vi "UHR-Fleezers Control (host) - 10.0.vi"() -> ()   [LabVIEW 2009] (continued)
        n1548 = Multiply(x=w7137, y=w7138) -> (x*y=w7136:dbl)
        n1549 = Divide(x=w7133, y=w7139) -> (x/y=w7132:dbl)
        n1550 = Divide(x=w7136, y=w7139) -> (x/y=w7135:dbl)
        n1551 = To Word Integer(number=w7132) -> (16bit integer=w7140:i16)
        n1552 = To Word Integer(number=w7135) -> (16bit integer=w7141:i16)
        n1553 = xnode "Read/Write Control"("FPGA VI Reference In"=w7131, "error in"=w7130, "AO1"=w7140, "AO2"=w7141) -> ("error out"=w7129:errorcluster)  [unwired: 1 out]
      }
      event #40 {
        n1554 = local read "Chemyx Syringe Pump Serial Port"() -> (w7197:refnum<visa-resource-name>)
        n1555 = event-data() -> ()  [unwired: 7 out]
        n1556 = local read "Pump write delay (ms)"() -> (w7198:dbl)
        n1557 = case shown="True" "Inject Pump 1" {
          tunnel: w7198 -> [w7205 w7219]
          tunnel: w7197 -> [w7202 w7218]
          frame #0 {
            n1558 = flat-sequence {
              tunnel: w7202 -> [w7206]
              tunnel: [w7206] -> w7203
              tunnel: w7205 -> [_]
              tunnel: [w7209] -> w7204
              tunnel: w7203 -> [w7209]
              tunnel: w7204 -> [w7210]
              tunnel: [w7210] -> w7200
              tunnel: [w7212] -> w7201
              tunnel: w7200 -> [w7212]
              tunnel: w7201 -> [w7214]
              frame #0 {
                n1559 = call "Write to pump.vi"("string"="enter pump1", "VISA resource name"=w7206) -> ()  [unwired: 1 out]
              }
              frame #1 {
                n1560 = Wait (ms)(milliseconds to wait="Pump pause delay (ms)") -> ()  [unwired: 1 out]
              }
              frame #2 {
                n1561 = call "Write to pump.vi"("string"="stop", "VISA resource name"=w7210) -> ()  [unwired: 1 out]
              }
              frame #3 {
                n1562 = Wait (ms)(milliseconds to wait=u32 500) -> ()  [unwired: 1 out]
              }
              frame #4 {
                n1563 = call "Write to pump.vi"("string"="stop", "VISA resource name"=w7214) -> ()  [unwired: 1 out]
              }
            }
          }
          frame #1 {
            n1564 = flat-sequence {
              tunnel: w7218 -> [w7228]
              tunnel: w7219 -> [w7223]
              tunnel: w7219 -> [w7230]
              tunnel: w7218 -> [w7231]
              tunnel: [w7231] -> w7216
              tunnel: [w7233] -> w7217
              tunnel: w7216 -> [w7233]
              tunnel: w7217 -> [w7235]
              frame #0 {
                n1565 = local read "All Pump Parameters"() -> (w7222:T5)
                n1566 = Unbundle By Name(w7222) -> ("Pump 1"=w7229:T45)
                n1567 = call "Set pump parameters.vi"("Pump write delay (ms)"=w7223, "Volume (uL)"="Ch 2 Inject Volume (uL)", "Rate (uL/h)"="Ch 1 Inject Rate (ul/h)", "Units"=4.0, "Pump #"=1.0, "Pump Parameters In"=w7229, "VISA resource name"=w7228) -> ("Pump Parameters Out"=w7221:T45)  [unwired: 3 in]
                n1568 = Bundle By Name(cluster=w7222, "Pump 1"=w7221) -> (w7220:T5)
                n1569 = local write "All Pump Parameters"(w7220) -> ()
              }
              frame #1 {
                n1570 = Wait (ms)(milliseconds to wait=w7230) -> ()  [unwired: 1 out]
              }
              frame #2 {
                n1571 = call "Write to pump.vi"("string"="start", "VISA resource name"=w7231) -> ()  [unwired: 1 out]
              }
              frame #3 {
                n1572 = Wait (ms)(milliseconds to wait=u32 500) -> ()  [unwired: 1 out]
              }
              frame #4 {
                n1573 = call "Write to pump.vi"("string"="start", "VISA resource name"=w7235) -> ()  [unwired: 1 out]
              }
            }
          }
        }
      }
      event #41 {
        n1574 = event-data() -> ()  [unwired: 7 out]
        n1575 = local read "Pump write delay (ms)"() -> (w7238:dbl)
        n1576 = case shown="False" "Inject Pump 3" {
          tunnel: w7238 -> [w7245 w7259]
          tunnel: "Chemyx Syringe Pump Serial Port" -> [w7242 w7258]
          frame #0 {
            n1577 = flat-sequence {
              tunnel: w7242 -> [w7246]
              tunnel: [w7246] -> w7243
              tunnel: w7245 -> [_]
              tunnel: [w7249] -> w7244
              tunnel: w7243 -> [w7249]
              tunnel: w7244 -> [w7250]
              tunnel: [w7250] -> w7240
              tunnel: [w7252] -> w7241
              tunnel: w7240 -> [w7252]
              tunnel: w7241 -> [w7254]
              frame #0 {
                n1578 = call "Write to pump.vi"("string"="enter pump3", "VISA resource name"=w7246) -> ()  [unwired: 1 out]
              }
              frame #1 {
                n1579 = local read "Pump pause delay (ms)"() -> (w7248:u32)
                n1580 = Wait (ms)(milliseconds to wait=w7248) -> ()  [unwired: 1 out]
              }
              frame #2 {
                n1581 = call "Write to pump.vi"("string"="stop", "VISA resource name"=w7250) -> ()  [unwired: 1 out]
              }
              frame #3 {
                n1582 = Wait (ms)(milliseconds to wait=u32 0) -> ()  [unwired: 1 out]
              }
              frame #4 {
                n1583 = call "Write to pump.vi"("string"="stop", "VISA resource name"=w7254) -> ()  [unwired: 1 out]
              }
            }
          }
          frame #1 {
            n1584 = flat-sequence {
              tunnel: w7258 -> [w7268]
              tunnel: w7259 -> [w7263]
              tunnel: w7259 -> [w7270]
              tunnel: w7258 -> [w7271]
              tunnel: [w7271] -> w7256
              tunnel: [w7274] -> w7257
              tunnel: w7256 -> [w7274]
              tunnel: w7257 -> [w7275]
              frame #0 {
                n1585 = local read "All Pump Parameters"() -> (w7262:T5)
                n1586 = Unbundle By Name(w7262) -> ("Pump 3"=w7269:T45)
                n1587 = call "Set pump parameters.vi"("Pump write delay (ms)"=w7263, "Volume (uL)"="Ch 3 Inject Volume (uL)", "Rate (uL/h)"="Ch 3 Inject Rate (ul/h)", "Units"=4.0, "Pump #"=3.0, "Pump Parameters In"=w7269, "VISA resource name"=w7268) -> ("Pump Parameters Out"=w7261:T45)  [unwired: 3 in]
                n1588 = Bundle By Name(cluster=w7262, "Pump 3"=w7261) -> (w7260:T5)
                n1589 = local write "All Pump Parameters"(w7260) -> ()
              }
              frame #1 {
                n1590 = Wait (ms)(milliseconds to wait=w7270) -> ()  [unwired: 1 out]
              }
              frame #2 {
                n1591 = call "Write to pump.vi"("string"="start", "VISA resource name"=w7271) -> ()  [unwired: 1 out]
              }
              frame #3 {
                n1592 = Wait (ms)(milliseconds to wait=u32 500) -> ()  [unwired: 1 out]
              }
              frame #4 {
                n1593 = call "Write to pump.vi"("string"="start", "VISA resource name"=w7275) -> ()  [unwired: 1 out]
              }
            }
          }
        }
      }
      event #42 {
        n1594 = event-data() -> ()  [unwired: 7 out]
        n1595 = local read "Pump write delay (ms)"() -> (w7279:dbl)
        n1596 = flat-sequence {
          tunnel: w7277 -> [w7292]
          tunnel: w7279 -> [w7288]
          tunnel: "Inject Pump 2" -> [_]
          tunnel: w7279 -> [w7294]
          tunnel: w7277 -> [w7295]
          frame #0 {
            n1597 = local read "All Pump Parameters"() -> (w7287:T5)
            n1598 = Multiply(x=60.0, y="Flush Center Ch Rate (ul/m)") -> (x*y=w7284:dbl)
            n1599 = Unbundle By Name(w7287) -> ("Pump 2"=w7293:T45)
            n1600 = call "Set pump parameters.vi"("Pump write delay (ms)"=w7288, "Volume (uL)"="Flush Center Ch Volume (uL)", "Rate (uL/h)"=w7284, "Units"=3.0, "Pump #"=2.0, "Pump Parameters In"=w7293, "VISA resource name"=w7292) -> ("Pump Parameters Out"=w7286:T45)  [unwired: 3 in]
            n1601 = Bundle By Name(cluster=w7287, "Pump 2"=w7286) -> (w7285:T5)
            n1602 = local write "All Pump Parameters"(w7285) -> ()
            n1603 = Add(x="Flush Center Ch Volume (uL)", y="Total Volume\nFlushed (uL)") -> (x+y=w7281:dbl)
            n1604 = local write "Total Volume\nFlushed (uL)"(w7281) -> ()
          }
          frame #1 {
            n1605 = Wait (ms)(milliseconds to wait=w7294) -> ()  [unwired: 1 out]
          }
          frame #2 {
            n1606 = call "Write to pump.vi"("string"="start", "VISA resource name"=w7295) -> ()  [unwired: 1 out]
          }
        }
        n1607 = local read "Chemyx Syringe Pump Serial Port"() -> (w7277:refnum<visa-resource-name>)
      }
      event #43 {
        n1608 = event-data() -> ()  [unwired: 7 out]
        n1609 = Select(t="run" ("string"), s="Sample Channel Flow", f="stop" ("string")) -> (s? t:f=w7297:string)
        n1610 = Concatenate Strings(w7297, "\r") -> (w7301:string)
        n1611 = VISA Write(VISA resource name=w7303, write buffer=w7301) -> ()  [unwired: 1 in, 3 out]
      }
      event #44 {
        n1612 = event-data() -> ()  [unwired: 7 out]
        n1613 = Not(x="Flip Green Filter") -> (.not. x?=w7304:bool)
        n1614 = local write "Flip Green Filter"(w7304) -> ()
        n1615 = flat-sequence {
          tunnel: w7312 -> [w7317]
          tunnel: w7311 -> [w7316]
          tunnel: [w7314] -> w7309
          tunnel: [w7313] -> w7308
          tunnel: [w7356] -> w7307
          tunnel: w7309 -> [w7356]
          tunnel: [w7355] -> w7306
          tunnel: w7308 -> [w7355]
          tunnel: w7307 -> [w7360]
          tunnel: w7306 -> [w7359]
          tunnel: [w7358] -> w7310
          frame #0 {
            n1616 = xnode "Read/Write Control"("FPGA VI Reference In"=w7317, "error in"=w7316, "Green Filter Flipper"=TRUE) -> ("FPGA VI Reference Out"=w7314:T20, "error out"=w7313:errorcluster)
          }
          frame #1 {
            n1617 = Wait (ms)(milliseconds to wait=u32 100) -> ()  [unwired: 1 out]
          }
          frame #2 {
            n1618 = xnode "Read/Write Control"("FPGA VI Reference In"=w7360, "error in"=w7359, "Green Filter Flipper"=FALSE) -> ("error out"=w7358:errorcluster)  [unwired: 1 out]
          }
        }
      }
      event #45 {
        n1619 = event-data() -> ()  [unwired: 7 out]
        n1620 = local read "Pump 1 contents"() -> (→"Pump 1 cont disp":string)
        n1621 = local read "Pump 3 contents"() -> (→"Pump 3 cont disp":string)
      }
      event #46 {
        n1622 = event-data() -> ()  [unwired: 7 out]
        n1623 = xnode "Read/Write Control"("FPGA VI Reference In"=w7403, "error in"=w7402, "Trap Pos. FB Reset"="Reset Trap Pos. FB") -> ()  [unwired: 2 out]
      }
      event #47 {
        n1624 = event-data() -> ()  [unwired: 7 out]
        n1625 = xnode "Read/Write Control"("FPGA VI Reference In"=w7443, "error in"=w7442, "Force feedback"="Trap Pos. FB ON") -> ()  [unwired: 2 out]
      }
      event #48 {
        n1626 = event-data() -> ()  [unwired: 7 out]
        n1627 = xnode "Read/Write Control"("FPGA VI Reference In"=w7489, "error in"=w7488, "Trap Pos. FB Range"="Trap Pos. FB Range", "Trap Pos. FB Gains"="Trap Pos. FB Gains", "Trap Pos. FB Mult Factor"="Trap Pos. FB Mult Factor", "Trap Pos. FB Offset Factor"="Trap Pos. FB Offset Factor", "Trap Pos FB Negate Action"="Trap Pos FB Negate Action", "Trap Pos FB Monitor T1 or T2"="Trap Pos FB Monitor\nT1 or T2", "AI1 X Scale"="Trap Pos. AI1 X Pre-scale") -> ()  [unwired: 2 out]
      }
      event #49 {
        n1628 = event-data() -> ()  [unwired: 7 out]
        n1629 = xnode "Read/Write Control"("FPGA VI Reference In"=w7625, "error in"=w7624, "Trap Pos. FB SP"="Trap Pos FB SP") -> ()  [unwired: 2 out]
      }
      event #50 {
        n1630 = event-data() -> ()  [unwired: 7 out]
        n1631 = local read "Trap Pos FB Monitor\nT1 or T2"() -> (w7677:bool)
        n1632 = local read "Trap X AI1 (DMA)"() -> (w7680:T10)
        n1633 = local read "Trap X AI1"() -> (w7683:T10)
        n1634 = Unbundle By Name(w7683) -> ("Set 1"=w7682:fxp<+/-,16,1>, "Set 2"=w7681:fxp<+/-,16,1>)
        n1635 = Unbundle By Name(w7680) -> ("Set 1"=w7679:fxp<+/-,16,1>, "Set 2"=w7678:fxp<+/-,16,1>)
        n1636 = Select(t=w7682, s=w7677, f=w7681) -> (s? t:f=w7676:fxp<+/-,16,1>)
        n1637 = Select(t=w7679, s=w7677, f=w7678) -> (s? t:f=w7675:fxp<+/-,16,1>)
        n1638 = Not(x="Set SP Using...") -> (.not. x?=w7670:bool)
        n1639 = Select(t=w7676, s=w7670, f=w7675) -> (s? t:f=w7671:fxp<+/-,16,1>)
        n1640 = xnode "Read/Write Control"("FPGA VI Reference In"=w7673, "error in"=w7672, "Trap Pos. FB SP"=w7671) -> ()  [unwired: 2 out]
        n1641 = local write "Trap Pos FB SP"(w7671) -> ()
      }
      event #51 {
        n1642 = event-data() -> ()  [unwired: 7 out]
        n1643 = Scale By Power Of 2(n="Trap Pos. FB Out Scale 2^n", x=ext 1.0) -> (x*2^n=w7729:ext)
        n1644 = property on="Trap Pos. FB Mult Factor" class="DigNum (strict)"("Val(Sgnl)"=w7729) -> ()  [unwired: 2 in, 2 out]
      }
    }
    "error out 2" <- w4459
    n1645 = node-c288() -> ()  [unwired: 2 out]
  }
  n1646 = timed-loop "Oscillate AOD (debugging)" {
    tunnel: w14 -> [w7733]
    tunnel: [w7732] -> w55
    timing: w50 -> [_]
    timing-out: [_] -> w49
    stop <- w7732 stop-if-true
    n1647 = node-c288() -> ()  [unwired: 2 out]
    n1648 = event shown="[0] \"Oscillate Set 1\", \"Fish for Tether\": Value Change" {
      selector: _ -> [_ _ _]
      dyn-events: _ -> [_ _ _]
      timeout: _ -> [_ _ _]
      tunnel: w7733 -> [w7740 _ _]
      tunnel: [FALSE ("Stop All") _ w7993] -> w7732
      event #0 {
        n1649 = event-data() -> ()  [unwired: 6 out]
        n1650 = local read "Oscillate Set 1"() -> (w7739:bool)
        n1651 = Or(x=w7739, y="Fish for Tether") -> (x .or. y?=w7737:bool)
        n1652 = case shown="True" w7737 {
          tunnel: w7740 -> [_ w7742]
          tunnel: "Fish for Tether" -> [_ w7741]
          frame #0 {
          }
          frame #1 {
            n1653 = case shown="True" w7741 {
              frame #0 {
              }
              frame #1 {
                n1654 = local write "Scan axis 2"(TRUE) -> ()
                n1655 = local write "Tether"(FALSE ("Tether")) -> ()
              }
            }
            n1656 = node-c288() -> (w7744:T22)  [unwired: 4 out]
            n1657 = timed-loop "Oscillate AOD" {
              timing: w7744 -> [_]
              timing-out: [_] -> w7743
              tunnel: w7742 -> [w7754]
              tunnel: w7741 -> [w7753]
              i -> [w7756]
              stop <- w7752 stop-if-true
              n1658 = node-c288() -> (w7755:i64)  [unwired: 1 out]
              n1659 = flat-sequence {
                tunnel: w7756 -> [w7783]
                tunnel: w7755 -> [w7782]
                tunnel: w7754 -> [w7761]
                tunnel: w7753 -> [w7764]
                tunnel: [w7764] -> w7751
                tunnel: [w7763] -> w7750
                tunnel: [w7760] -> w7749
                tunnel: [w7757] -> w7747
                tunnel: w7751 -> [w7819]
                tunnel: w7750 -> [w7817]
                tunnel: w7749 -> [w7816]
                tunnel: [w7815] -> w7748
                tunnel: w7747 -> [w7814]
                tunnel: [w7867] -> w7752
                tunnel: w7748 -> [w7866]
                frame #0 {
                  n1660 = Divide(x=w7782, y=i64 1000) -> (x/y=w7777:dbl)
                  n1661 = Multiply(x=w7777, y=w7783) -> (x*y=w7779:dbl)
                  n1662 = local read "BD 1 Frequency 2 (MHz)"() -> (w7762:dbl)
                  n1663 = Multiply(x="Osc. freq. (Hz)", y=6.283185307179586) -> (x*y=w7780:dbl)
                  n1664 = Multiply(x=w7780, y=w7779) -> (x*y=w7759:dbl)
                  n1665 = local read "BD 1 Frequency 1 (MHz)"() -> (w7767:dbl)
                  n1666 = case shown="True" w7764 {
                    tunnel: w7759 -> [w7789 w7794]
                    tunnel: w7767 -> [_ w7805]
                    tunnel: w7762 -> [_ w7806]
                    tunnel: [w7786 w7800] -> w7765
                    tunnel: [FALSE w7797] -> w7760
                    tunnel: [0.0 w7790] -> w7757
                    frame #0 {
                      n1667 = Sine(x=w7789) -> (sin(x)=w7787:dbl)
                      n1668 = Multiply(x=w7787, y="Osc. amp. (MHz)") -> (x*y=w7786:dbl)
                    }
                    frame #1 {
                      n1669 = Cosine(x=w7794) -> (cos(x)=w7809:dbl)
                      n1670 = Subtract(x=w7806, y=w7805) -> (x-y=w7804:dbl)
                      n1671 = Decrement(x=w7809) -> (x-1=w7808:dbl)
                      n1672 = Subtract(x=w7804, y="Closest Delta (MHz)") -> (x-y=w7801:dbl)
                      n1673 = Divide(x=w7808, y=-2.0) -> (x/y=w7802:dbl)
                      n1674 = Multiply(x=w7802, y=w7801) -> (x*y=w7800:dbl)
                      n1675 = local read "Vec Mean of T1 T2"() -> (w7796:dbl[])
                      n1676 = Greater?(x=w7796, y="Stop F (pN)") -> (0:w7798:bool[])
                      n1677 = Or Array Elements(Boolean array=w7798) -> (logical OR=w7797:bool)
                      n1678 = Divide(x=w7794, y=6.283185307179586) -> (x/y=w7793:dbl)
                      n1679 = Round Toward +Infinity(x=w7793) -> (ceil(x): smallest int >= x=w7790:dbl)
                      "Attempts" <- w7790
                      n1680 = Greater?(x=w7790, y="Attempt Limit") -> (0:w7792:bool)
                      n1681 = case shown="True" w7792 {
                        frame #0 {
                        }
                        frame #1 {
                          n1682 = call <vilib>:"Beep.vi"() -> ()  [unwired: 3 in, 9 out]
                          n1683 = local write "Fish for Tether"(FALSE ("Fish for Tether")) -> ()
                          n1684 = local read "Messages"() -> (w7811:string)
                          n1685 = call "Update messages.vi"("Message to add"="Tether fishing timeout." ("Messages"), "Old message string"=w7811) -> ("New message string"=→"Messages":string)
                        }
                      }
                    }
                  }
                  n1686 = local read "BD 2 Frequency 1 (MHz)"() -> (w7766:dbl)
                  n1687 = Select(t=w7767, s="Scan axis 2", f=w7766) -> (s? t:f=w7770:dbl)
                  n1688 = Add(x=w7765, y=w7770) -> (x+y=w7763:dbl)
                  n1689 = Select(t=w7763, s="Scan axis 2", f=w7767) -> (s? t:f=w7773:dbl)
                  n1690 = Select(t=w7766, s="Scan axis 2", f=w7763) -> (s? t:f=w7772:dbl)
                  n1691 = local read "Y RF Frequency Limits (MHz)"() -> (w7768:T15)
                  n1692 = local read "X RF Frequency Limits (MHz)"() -> (w7769:T15)
                  n1693 = local read "BD 1 Frequency 3 (MHz)"() -> (w7776:dbl)
                  n1694 = local read "BD 2 Frequency 2 (MHz)"() -> (w7775:dbl)
                  n1695 = local read "BD 2 Frequency 3 (MHz)"() -> (w7774:dbl)
                  n1696 = call "set RF board frequency - interlace.vi"("Board 2 Frequency Limits"=w7768, "Board 1 Frequency Limits"=w7769, "FPGA VI Reference In"=w7761, "Board 2 Frequency 3 (MHz)"=w7774, "Board 1 Frequency 3 (MHz)"=w7776, "Board 2 Frequency 2 (MHz)"=w7775, "Board 2 Frequency 1 (MHz)"=w7772, "Board 1 Frequency 2 (MHz)"=w7762, "Board 1 Frequency 1  (MHz)"=w7773) -> ()  [unwired: 1 in, 2 out]
                }
                frame #1 {
                  n1697 = And(x=w7819, y=w7816) -> (x .and. y?=w7818:bool)
                  n1698 = case "Only if were fishing and now formed tether" shown="True" w7818 {
                    tunnel: w7817 -> [w7821 w7834]
                    tunnel: [w7820 w7833] -> w7815
                    tunnel: w7814 -> [_ w7829]
                    frame #0 {
                      n1699 = local read "Fish for Tether"() -> (w7820:bool)
                      n1700 = case shown="False" w7820 {
                        tunnel: w7821 -> [w7822 _]
                        frame #0 {
                          n1701 = property on="BD 1 Frequency 1 (MHz)" class="DigNum (strict)"("Val(Sgnl)"=w7822) -> ()  [unwired: 2 in, 2 out]
                        }
                        frame #1 {
                        }
                      }
                    }
                    frame #1 {
                      w7833 = FALSE ("Fish for Tether")
                      n1702 = call <vilib>:"Beep.vi"() -> ()  [unwired: 3 in, 9 out]
                      n1703 = Number To Decimal String(number=w7829, width (-)=i16 1) -> (decimal integer string=w7827:string)
                      n1704 = case shown="\"2\", \"3\", \"4\", \"5\", \"6\"" "Then..." {
                        selector: "Then..." -> [_ w7837]
                        tunnel: w7834 -> [w7836 _]
                        frame #0 {
                          n1705 = property on="BD 1 Frequency 1 (MHz)" class="DigNum (strict)"("Val(Sgnl)"=w7836) -> ()  [unwired: 2 in, 2 out]
                        }
                        frame #1 {
                          n1706 = flat-sequence {
                            tunnel: w7837 -> [w7839]
                            frame #0 {
                              n1707 = property on="Trap Delta (MHz)" class="DigNum (strict)"("Val(Sgnl)"="Move to Delta 1 (MHz)") -> ()  [unwired: 2 in, 2 out]
                            }
                            frame #1 {
                              n1708 = case shown="\"5\", \"6\"" w7839 {
                                selector: w7839 -> [w7842 w7852 _]
                                frame #0 {
                                n1709 = flat-sequence {
                                tunnel: w7842 -> [w7843]
                                tunnel: [w7843] -> w7840
                                tunnel: [w7845] -> w7841
                                tunnel: w7840 -> [w7845]
                                tunnel: w7841 -> [w7849]
                                frame #0 {
                                n1710 = property on="Green Laser ON/Interlacing" class="Bool (strict)"("Val(Sgnl)"=TRUE ("Value (Signaling)")) -> ()  [unwired: 2 in, 2 out]
                                }
                                frame #1 {
                                n1711 = Multiply(x="Wait Before Save (s)", y=u32 1000 ("x")) -> (x*y=w7847:u32)
                                n1712 = Wait (ms)(milliseconds to wait=w7847) -> ()  [unwired: 1 out]
                                }
                                frame #2 {
                                n1713 = property on="Start Saving" class="Bool (strict)"("Value"=TRUE ("Start Saving")) -> ()  [unwired: 2 in, 2 out]
                                n1714 = case shown="\"4\"" w7849 {
                                frame #0 {
                                }
                                frame #1 {
                                n1715 = property on="Fl. Triggered..." class="Bool (strict)"("Val(Sgnl)"=TRUE ("Value (Signaling)")) -> ()  [unwired: 2 in, 2 out]
                                }
                                }
                                }
                                }
                                }
                                frame #1 {
                                n1716 = flat-sequence {
                                tunnel: w7852 -> [w7860]
                                frame #0 {
                                n1717 = Wait (ms)(milliseconds to wait=u32 500) -> ()  [unwired: 1 out]
                                }
                                frame #1 {
                                n1718 = property on="Trap Raster Scan" class="Bool (strict)"("Val(Sgnl)"=TRUE ("Value (Signaling)")) -> ()  [unwired: 2 in, 2 out]
                                }
                                frame #2 {
                                n1719 = Wait (ms)(milliseconds to wait=u32 500) -> ()  [unwired: 1 out]
                                }
                                frame #3 {
                                n1720 = while {
                                stop <- w7856 stop-if-true
                                n1721 = local read "Saving..."() -> (w7857:bool)
                                n1722 = Wait (ms)(milliseconds to wait=u32 100) -> ()  [unwired: 1 out]
                                n1723 = Not(x=w7857) -> (.not. x?=w7856:bool)
                                }
                                }
                                frame #4 {
                                n1724 = property on="Trap Delta (MHz)" class="DigNum (strict)"("Val(Sgnl)"="Move to Delta 2 (MHz)") -> ()  [unwired: 2 in, 2 out]
                                }
                                frame #5 {
                                n1725 = case shown="\"6\"" w7860 {
                                frame #0 {
                                }
                                frame #1 {
                                n1726 = local read "Tether"() -> (w7861:bool)
                                n1727 = case shown="True" w7861 {
                                frame #0 {
                                }
                                frame #1 {
                                n1728 = flat-sequence {
                                frame #0 {
                                n1729 = Wait (ms)(milliseconds to wait=u32 500) -> ()  [unwired: 1 out]
                                }
                                frame #1 {
                                n1730 = property on="Green Laser ON/Interlacing" class="Bool (strict)"("Val(Sgnl)"=TRUE ("Green Laser ON/Interlacing")) -> ()  [unwired: 2 in, 2 out]
                                }
                                frame #2 {
                                n1731 = Wait (ms)(milliseconds to wait=u32 500) -> ()  [unwired: 1 out]
                                }
                                frame #3 {
                                n1732 = local write "Start Saving"(TRUE ("Start Saving")) -> ()
                                }
                                }
                                }
                                }
                                }
                                }
                                }
                                }
                                }
                                frame #2 {
                                }
                              }
                            }
                          }
                        }
                      }
                      n1733 = Concatenate Strings("Formed tether in ", w7827, " attempt(s)." ("string")) -> (w7824:string)
                      n1734 = local read "Messages"() -> (w7831:string)
                      n1735 = local write "Fish for Tether"(w7833) -> ()
                      n1736 = call "Update messages.vi"("Message to add"=w7824, "Old message string"=w7831) -> ("New message string"=w7830:string)
                      n1737 = local write "Messages"(w7830) -> ()
                      n1738 = Get Date/Time In Seconds() -> (seconds since 1Jan1904=→"Time tether formed":timestamp)
                      "Tether" <- "Tether Alarm?"
                    }
                  }
                }
                frame #2 {
                  n1739 = local read "Oscillate Set 1"() -> (w7871:bool)
                  n1740 = Or(x=w7871, y=w7866) -> (x .or. y?=w7868:bool)
                  n1741 = local read "Stop All"() -> (w7869:bool)
                  n1742 = Not(x=w7868) -> (.not. x?=w7870:bool)
                  n1743 = Compound Arithmetic op=OR(w7869, w7870) -> (w7867:bool)
                }
              }
              n1744 = node-c288() -> ()  [unwired: 2 out]
            }
            n1745 = node-c288(w7743) -> ()  [unwired: 1 out]
          }
        }
      }
      event #1 {
        n1746 = event-data() -> ()  [unwired: 7 out]
        n1747 = case shown="True" "Fl. Triggered..." {
          frame #0 {
          }
          frame #1 {
            n1748 = node-c288() -> (w7881:T22)  [unwired: 4 out]
            n1749 = timed-loop {
              timing: w7881 -> [_]
              timing-out: [_] -> w7880
              tunnel: "Action" -> [w7885]
              shift-right: [w7882] -> _
              shift-left: u8 255 -> [w7884]
              stop <- w7886 stop-if-true
              n1750 = node-c288() -> ()  [unwired: 2 out]
              n1751 = flat-sequence {
                tunnel: w7885 -> [w7898]
                tunnel: w7884 -> [w7895]
                tunnel: [w7894] -> w7883
                tunnel: [w7984] -> w7886
                tunnel: w7883 -> [w7983]
                tunnel: [w7983] -> w7882
                frame #0 {
                  n1752 = local read "Delta Fl. 2"() -> (w7889:dbl)
                  n1753 = local read "Delta Fl. 1"() -> (w7890:dbl)
                  n1754 = Select(t=w7890, s="APD to Watch", f=w7889) -> (s? t:f=w7888:dbl)
                  n1755 = Multiply(x="Fl. Delta Thresh. (kHz)", y=1000.0) -> (x*y=w7897:dbl)
                  n1756 = Greater?(x=w7888, y=w7897) -> (0:w7892:bool)
                  n1757 = Or(x="Force Yank", y=w7892) -> (x .or. y?=w7893:bool)
                  n1758 = case shown="True" w7893 {
                    tunnel: w7898 -> [_ w7908]
                    tunnel: w7895 -> [w7900 w7904]
                    tunnel: [w7900 w7901] -> w7894
                    frame #0 {
                    }
                    frame #1 {
                      n1759 = flat-sequence {
                        tunnel: w7905 -> [w7914]
                        tunnel: [w7914] -> w7909
                        tunnel: w7908 -> [w7913]
                        tunnel: [w7913] -> w7907
                        tunnel: [w7912] -> w7906
                        tunnel: w7904 -> [w7911]
                        tunnel: [w7910] -> w7903
                        tunnel: w7909 -> [w7939]
                        tunnel: w7907 -> [w7938]
                        tunnel: w7906 -> [w7937]
                        tunnel: w7903 -> [w7936]
                        tunnel: [w7936] -> w7902
                        tunnel: w7902 -> [w7981]
                        tunnel: [w7981] -> w7901
                        frame #0 {
                          n1760 = call <vilib>:"Beep.vi"() -> ()  [unwired: 3 in, 9 out]
                          n1761 = local write "Waiting"(FALSE ("Waiting")) -> ()
                          n1762 = Increment(x=w7911) -> (x+1=w7910:u8)
                          n1763 = case shown="\"Yank\"" w7913 {
                            tunnel: w7910 -> [_ _ w7920]
                            frame #0 {
                              n1764 = property on="Confocal Image" class="Bool (strict)"("Val(Sgnl)"=TRUE ("Value (Signaling)")) -> ()  [unwired: 2 in, 2 out]
                            }
                            frame #1 {
                            }
                            frame #2 {
                              n1765 = flat-sequence {
                                tunnel: w7920 -> [w7923]
                                tunnel: [w7922] -> w7919
                                tunnel: ["N Array El"] -> w7918
                                tunnel: w7919 -> [w7933]
                                tunnel: w7918 -> [w7929]
                                frame #0 {
                                n1766 = Multiply(x="Yank Delay (s)", y=1000.0) -> (x*y=w7926:dbl)
                                n1767 = Quotient & Remainder(x=w7923, y="N Array El") -> (x-y*floor(x/y)=w7922:u8)  [unwired: 1 out]
                                n1768 = Wait (ms)(milliseconds to wait=w7926) -> ()  [unwired: 1 out]
                                }
                                frame #1 {
                                n1769 = Random Number (0-1)() -> (number: 0 to 1=w7930:dbl)
                                n1770 = Multiply(x=w7929, y=w7930) -> (x*y=w7928:dbl)
                                n1771 = Round Toward -Infinity(1:w7928) -> (0:w7927:dbl)
                                n1772 = Select(t=w7927, s="Random Choice", f=w7933) -> (s? t:f=w7931:dbl)
                                n1773 = Index Array(array="Yank to Delta Array (MHz)", index=w7931) -> (element=w7934:dbl)
                                n1774 = property on="Trap Delta (MHz)" class="DigNum (strict)"("Val(Sgnl)"=w7934) -> ()  [unwired: 2 in, 2 out]
                                }
                              }
                            }
                          }
                          n1775 = local read "Time (s)"() -> (w7912:dbl)
                          "Fl. High" <- TRUE ("Yanking")
                        }
                        frame #1 {
                          n1776 = node-c288() -> (w7941:T22)  [unwired: 4 out]
                          n1777 = timed-loop {
                            timing: w7941 -> [_]
                            timing-out: [_] -> w7940
                            tunnel: w7939 -> [w7957]
                            tunnel: w7938 -> [w7955]
                            tunnel: w7937 -> [w7954]
                            stop <- w7956 stop-if-true
                            n1778 = node-c288() -> ()  [unwired: 2 out]
                            n1779 = local read "Fl. Delta Thresh. (kHz)"() -> (w7949:dbl)
                            n1780 = local read "Fl. Triggered..."() -> (w7958:bool)
                            n1781 = local read "Delta Fl. 1"() -> (w7945:dbl)
                            n1782 = local read "Delta Fl. 2"() -> (w7943:dbl)
                            n1783 = local read "Stop All"() -> (w7952:bool)
                            n1784 = local read "APD to Watch"() -> (w7944:bool)
                            n1785 = Select(t=w7945, s=w7944, f=w7943) -> (s? t:f=w7942:dbl)
                            n1786 = Not(x=w7958) -> (.not. x?=w7953:bool)
                            n1787 = Multiply(x=w7949, y=1000.0) -> (x*y=w7948:dbl)
                            n1788 = Negate(x=w7948) -> (-x=w7947:dbl)
                            n1789 = Less?(x=w7942, y=w7947) -> (x < y?=w7951:bool)
                            n1790 = Compound Arithmetic op=OR(w7951, w7952, w7953, "Force Reset") -> (w7956:bool)
                            n1791 = case shown="True" w7956 {
                              tunnel: w7957 -> [_ w7969]
                              tunnel: w7955 -> [_ w7968]
                              tunnel: w7954 -> [_ w7966]
                              frame #0 {
                              }
                              frame #1 {
                                n1792 = case shown="\"Yank\"" w7968 {
                                tunnel: w7969 -> [_ w7970]
                                frame #0 {
                                }
                                frame #1 {
                                n1793 = flat-sequence {
                                tunnel: [w7975] -> w7971
                                tunnel: w7970 -> [w7975]
                                tunnel: w7971 -> [w7976]
                                frame #0 {
                                n1794 = local read "Yank Delay (s)"() -> (w7974:dbl)
                                n1795 = Multiply(x=w7974, y=1000.0) -> (x*y=w7972:dbl)
                                n1796 = Wait (ms)(milliseconds to wait=w7972) -> ()  [unwired: 1 out]
                                }
                                frame #1 {
                                n1797 = property on="Trap Delta (MHz)" class="DigNum (strict)"("Val(Sgnl)"=w7976) -> ()  [unwired: 2 in, 2 out]
                                }
                                }
                                }
                                }
                                n1798 = local read "Time (s)"() -> (w7967:dbl)
                                n1799 = Subtract(x=w7967, y=w7966) -> (x-y=w7963:dbl)
                                "Duration (s)" <- w7963
                                n1800 = Number To Decimal String(number=w7963, width (-)=i16 0) -> (decimal integer string=w7961:string)
                                n1801 = Concatenate Strings(w7961, " s fluorescence event." ("string")) -> (w7959:string)
                                n1802 = local read "Messages"() -> (w7965:string)
                                n1803 = call "Update messages.vi"("Message to add"=w7959, "Old message string"=w7965) -> ("New message string"=w7964:string)
                                n1804 = call <vilib>:"Beep.vi"() -> ()  [unwired: 3 in, 9 out]
                                n1805 = local write "Messages"(w7964) -> ()
                              }
                            }
                            n1806 = node-c288() -> ()  [unwired: 2 out]
                          }
                          n1807 = node-c288(w7940) -> ()  [unwired: 1 out]
                        }
                        frame #2 {
                          n1808 = local write "Fl. High"(FALSE ("Yanking")) -> ()
                        }
                      }
                      n1809 = local read "Trap Delta (MHz)"() -> (w7905:dbl)
                    }
                  }
                }
                frame #1 {
                  n1810 = local read "Stop All"() -> (w7987:bool)
                  n1811 = local read "Fl. Triggered..."() -> (w7985:bool)
                  n1812 = Not(x=w7985) -> (.not. x?=w7986:bool)
                  n1813 = Or(x=w7986, y=w7987) -> (x .or. y?=w7984:bool)
                  n1814 = Not(x=w7984) -> (.not. x?=→"Waiting":bool)
                }
              }
              n1815 = node-c288() -> ()  [unwired: 2 out]
            }
            n1816 = node-c288(w7880) -> ()  [unwired: 1 out]
          }
        }
      }
      event #2 {
        n1817 = event-data() -> ()  [unwired: 7 out]
        n1818 = local read "Stop All"() -> (w7993:bool)
      }
    }
    n1819 = node-c288() -> ()  [unwired: 2 out]
  }
  n1820 = timed-loop "Mouse control: trap position (AOM deflection), set confocal spot from image" {
    tunnel: [w7995] -> w164
    tunnel: w14 -> [w7994]
    timing: w54 -> [_]
    timing-out: [_] -> w53
    stop <- w7995 stop-if-true
    n1821 = node-c288() -> ()  [unwired: 2 out]
    n1822 = event shown="[0] \"Pane\": Mouse Down" {
      selector: _ -> [_ _]
      dyn-events: _ -> [_ _]
      timeout: _ -> [_ _]
      tunnel: w7994 -> [w7998 _]
      event #0 {
        n1823 = event-data() -> ("Time"=w8000:u32, "Coords"=w7999:T7, "Button"=w8001:u16)  [unwired: 6 out]
        n1824 = case shown="1" w8001 {
          tunnel: w8000 -> [_ _ w8104]
          tunnel: w7999 -> [_ w8038 w8102]
          tunnel: w7998 -> [_ _ w8100]
          frame #0 {
          }
          frame #1 {
            n1825 = property on="APD 2" class="ImageControl"() -> ("Displayed Image Position"=w8008:cluster{"Left":i32, "Top":i32})  [unwired: 2 in, 2 out]
            n1826 = property on="APD 1" class="ImageControl"() -> ("Displayed Image Position"=w8037:cluster{"Left":i32, "Top":i32})  [unwired: 2 in, 2 out]
            n1827 = property on="Detection Laser X" class="ImageControl"() -> ("Displayed Image Position"=w8034:cluster{"Left":i32, "Top":i32})  [unwired: 2 in, 2 out]
            n1828 = property on="Detection Laser Y" class="ImageControl"() -> ("Displayed Image Position"=w8033:cluster{"Left":i32, "Top":i32})  [unwired: 2 in, 2 out]
            n1829 = property on="APD 2" class="ImageControl"() -> ("Displayed Image Size"=w8007:cluster{"Width":u32, "Height":u32})  [unwired: 2 in, 2 out]
            n1830 = property on="APD 1" class="ImageControl"() -> ("Displayed Image Size"=w8035:cluster{"Width":u32, "Height":u32})  [unwired: 2 in, 2 out]
            n1831 = property on="Detection Laser X" class="ImageControl"() -> ("Displayed Image Size"=w8036:cluster{"Width":u32, "Height":u32})  [unwired: 2 in, 2 out]
            n1832 = property on="Detection Laser Y" class="ImageControl"() -> ("Displayed Image Size"=w8032:cluster{"Width":u32, "Height":u32})  [unwired: 2 in, 2 out]
            n1833 = Unbundle By Name(w8007) -> ("Width"=w8004:u32, "Height"=w8003:u32)
            n1834 = Unbundle By Name(w8008) -> ("Left"=w8006:i32, "Top"=w8005:i32)
            n1835 = Unbundle By Name(w8035) -> ("Width"=w8029:u32, "Height"=w8028:u32)
            n1836 = Unbundle By Name(w8036) -> ("Width"=w8025:u32, "Height"=w8024:u32)
            n1837 = Unbundle By Name(w8032) -> ("Width"=w8021:u32, "Height"=w8020:u32)
            n1838 = Unbundle By Name(w8037) -> ("Left"=w8031:i32, "Top"=w8030:i32)
            n1839 = Unbundle By Name(w8034) -> ("Left"=w8027:i32, "Top"=w8026:i32)
            n1840 = Unbundle By Name(w8033) -> ("Left"=w8023:i32, "Top"=w8022:i32)
            n1841 = Bundle("Left"=w8006, "Top"=w8005, "Width"=w8004, "Height"=w8003) -> (w8002:T46)  [unwired: 1 in]
            n1842 = Bundle("Left"=w8031, "Top"=w8030, "Width"=w8029, "Height"=w8028) -> (w8019:T46)  [unwired: 1 in]
            n1843 = Bundle("Left"=w8027, "Top"=w8026, "Width"=w8025, "Height"=w8024) -> (w8018:T46)  [unwired: 1 in]
            n1844 = Bundle("Left"=w8023, "Top"=w8022, "Width"=w8021, "Height"=w8020) -> (w8017:T46)  [unwired: 1 in]
            n1845 = Build Cluster Array(w8002, w8019, w8018, w8017) -> (w8016:T47)
            n1846 = for {
              tunnel: w8038 -> [w8049]
              tunnel: w8016 -> [w8050] mode=indexing
              shift-right: [w8047] -> w8014
              shift-left: TRUE -> [w8048]
              shift-right: [w8046] -> w8012
              shift-left: _ -> [w8042]
              shift-right: [w8045] -> w8011
              shift-left: _ -> [w8041]
              shift-right: [w8044] -> w8010
              shift-left: _ -> [w8040]
              shift-right: [w8043] -> w8009
              shift-left: _ -> [w8039]
              n1847 = case shown="True" w8048 {
                selector: w8048 -> [w8055 _]
                tunnel: w8050 -> [_ w8064]
                tunnel: w8049 -> [_ w8062]
                tunnel: [w8055 w8060] -> w8047
                tunnel: [w8054 w8059] -> w8046
                tunnel: [w8053 w8058] -> w8045
                tunnel: [w8052 w8057] -> w8044
                tunnel: [w8051 w8056] -> w8043
                tunnel: w8042 -> [w8054 _]
                tunnel: w8041 -> [w8053 _]
                tunnel: w8040 -> [w8052 _]
                tunnel: w8039 -> [w8051 _]
                frame #0 {
                }
                frame #1 {
                  n1848 = Unbundle(w8064) -> (w8063:T46)
                  n1849 = call "isclickinwindow.vi"("Image Param"=w8063, "Point32"=w8062) -> ("4 Y"=w8056:i32, "3 Height"=w8057:i32, "2 X"=w8058:i32, "1 Width"=w8059:i32, "In image?"=w8061:bool)  [unwired: 1 in]
                  n1850 = Not(x=w8061) -> (.not. x?=w8060:bool)
                }
              }
            }
            n1851 = Not(x=w8014) -> (.not. x?=w8013:bool)
            n1852 = case shown="True" w8013 {
              tunnel: w8011 -> [_ w8077]
              tunnel: w8009 -> [_ w8076]
              tunnel: w8012 -> [_ w8075]
              tunnel: w8010 -> [_ w8074]
              frame #0 {
              }
              frame #1 {
                w8070 = FALSE ("Get Point")
                n1853 = local read "Scan lines (y)"() -> (w8079:u64)
                n1854 = local read "Actual MCL Inc (V)"() -> (w8071:dbl)
                n1855 = local read "Scan steps (MCL)"() -> (w8078:u64)
                n1856 = Divide "Y Pix/step"(x=w8074, y=w8079) -> (x/y=w8086:dbl)
                n1857 = Divide "Y V/pix"(x=w8071, y=w8086) -> (x/y=w8085:dbl)
                n1858 = Divide "Y half step offset"(x=w8071, y=2.0) -> (x/y=w8087:dbl)
                n1859 = Divide "X pix/step"(x=w8075, y=w8078) -> (x/y=w8084:dbl)
                n1860 = Negate(x=w8087) -> (-x=w8088:dbl)
                n1861 = local read "Initial Y"() -> (w8094:dbl)
                n1862 = Multiply(x=w8076, y=w8085) -> (x*y=w8095:dbl)
                n1863 = Divide "X half step offset"(x=w8071, y=2.0) -> (x/y=w8081:dbl)
                n1864 = Divide "X V/pix"(x=w8071, y=w8084) -> (x/y=w8083:dbl)
                n1865 = Multiply(x=w8071, y=w8078) -> (x*y=w8090:dbl)
                n1866 = Compound Arithmetic op=ADD(w8088, w8095, w8094) -> (w8072:dbl)
                "Pointer Y (V)" <- w8072
                n1867 = Multiply(x=w8083, y=w8077) -> (x*y=w8092:dbl)
                n1868 = Negate(x=w8081) -> (-x=w8080:dbl)
                n1869 = local read "Initial X"() -> (w8093:dbl)
                n1870 = Negate(x=w8092) -> (-x=w8091:dbl)
                n1871 = Compound Arithmetic op=ADD(w8080, w8090, w8093, w8091) -> (w8073:dbl)
                "Pointer X (V)" <- w8073
                n1872 = Or(x="Set X Only", y="Set Confocal Spot (X-Y)") -> (x .or. y?=w8066:bool)
                n1873 = Or(x="Set Confocal Spot (X-Y)", y="Set Y Only") -> (x .or. y?=w8065:bool)
                n1874 = case shown="True" w8066 {
                  tunnel: w8073 -> [_ w8096]
                  frame #0 {
                  }
                  frame #1 {
                    n1875 = property on="AO2" class="Slide (strict)"("Val(Sgnl)"=w8096) -> ()  [unwired: 2 in, 2 out]
                  }
                }
                n1876 = case shown="True" w8065 {
                  tunnel: w8072 -> [_ w8097]
                  frame #0 {
                  }
                  frame #1 {
                    n1877 = property on="AO1" class="Slide (strict)"("Val(Sgnl)"=w8097) -> ()  [unwired: 2 in, 2 out]
                  }
                }
                n1878 = local write "Set Confocal Spot (X-Y)"(w8070) -> ()
                n1879 = local write "Set X Only"(w8070) -> ()
                n1880 = local write "Set Y Only"(w8070) -> ()
              }
            }
          }
          frame #2 {
            n1881 = local read "BD 2 Frequency 1 (MHz)"() -> (w8098:dbl)
            n1882 = local read "BD 1 Frequency 1 (MHz)"() -> (w8099:dbl)
            n1883 = local write "Manipulating Trap"(TRUE ("Manipulating Trap")) -> ()
            n1884 = local write "Coords"(T7 {"Horizontal"=0, "Vertical"=0} ("Coords")) -> ()
            n1885 = while {
              tunnel: w8104 -> [w8109]
              tunnel: w8102 -> [w8108]
              tunnel: w8100 -> [w8107]
              tunnel: w8099 -> [w8106]
              tunnel: w8098 -> [w8105]
              stop <- w8110 stop-if-true
              n1886 = event shown="[0] \"Pane\": Mouse Move" {
                selector: _ -> [_ _]
                dyn-events: _ -> [_ _]
                timeout: _ -> [_ _]
                tunnel: ["Force Manip Abort" w8174] -> w8110
                tunnel: w8109 -> [w8117 _]
                tunnel: w8108 -> [w8115 _]
                tunnel: w8107 -> [w8114 _]
                tunnel: w8106 -> [w8113 _]
                tunnel: w8105 -> [w8112 _]
                event #0 {
                  n1887 = event-data() -> ("Time"=w8118:u32, "Coords"=w8119:T7)  [unwired: 3 out]
                  n1888 = Less?(x=w8118, y=w8117) -> (x < y?=w8116:bool)
                  n1889 = case "Makes sure old motion events prior to mouse click aren't used" shown="False" w8116 {
                    tunnel: w8119 -> [w8161 _]
                    tunnel: w8115 -> [w8162 _]
                    tunnel: w8114 -> [w8139 _]
                    tunnel: w8113 -> [w8135 _]
                    tunnel: w8112 -> [w8134 _]
                    frame #0 {
                      n1890 = Subtract(x=w8161, y=w8162) -> (x-y=w8160:T7)
                      "Coords" <- w8160
                      n1891 = local read "Y RF Frequency Limits (MHz)"() -> (w8120:T15)
                      n1892 = To Double Precision Float(number=w8160) -> (double precision float=w8159:cluster{"Horizontal":dbl, "Vertical":dbl})
                      n1893 = Multiply(x=cluster{"Horizontal":dbl, "Vertical":dbl} {"Horizontal"=-1.0, "Vertical"=1.0}, y="Manipulation Scaling") -> (x*y=w8155:cluster{"Horizontal":dbl, "Vertical":dbl})
                      n1894 = local read "X RF Frequency Limits (MHz)"() -> (w8121:T15)
                      n1895 = Multiply(x=w8159, y=w8155) -> (x*y=w8157:cluster{"Horizontal":dbl, "Vertical":dbl})
                      n1896 = Unbundle By Name(w8157) -> ("Horizontal"=w8152:dbl, "Vertical"=w8156:dbl)
                      n1897 = Unbundle By Name(w8120) -> ("Maximum"=w8123:dbl, "Minimum"=w8122:dbl)
                      n1898 = Boolean To (0,1)(Boolean="Manip. X?") -> (0, 1=w8150:i16)
                      n1899 = Boolean To (0,1)(Boolean="Manip. Y?") -> (0, 1=w8147:i16)
                      n1900 = Multiply(x=w8156, y=w8147) -> (x*y=w8149:dbl)
                      n1901 = Multiply(x=w8150, y=w8152) -> (x*y=w8153:dbl)
                      n1902 = local read "BD 1 Frequency 2 (MHz)"() -> (w8137:dbl)
                      n1903 = Unbundle By Name(w8121) -> ("Maximum"=w8125:dbl, "Minimum"=w8124:dbl)
                      n1904 = local read "BD 2 Frequency 2 (MHz)"() -> (w8136:dbl)
                      n1905 = Add(x=w8134, y=w8149) -> (x+y=w8127:dbl)
                      n1906 = Add(x=w8135, y=w8153) -> (x+y=w8129:dbl)
                      n1907 = In Range and Coerce(upper limit=w8125, x=w8129, lower limit=w8124) -> (coerced(x)=w8128:dbl)  [unwired: 1 out]
                      n1908 = In Range and Coerce(upper limit=w8123, x=w8127, lower limit=w8122) -> (coerced(x)=w8126:dbl)  [unwired: 1 out]
                      n1909 = Subtract(x=w8128, y=w8137) -> (x-y=w8146:dbl)
                      n1910 = Subtract(x=w8126, y=w8136) -> (x-y=w8145:dbl)
                      n1911 = Square(x=w8146) -> (x^2=w8144:dbl)
                      n1912 = Square(x=w8145) -> (x^2=w8143:dbl)
                      n1913 = Add(x=w8144, y=w8143) -> (x+y=w8142:dbl)
                      n1914 = Square Root(x=w8142) -> (sqrt(x)=w8138:dbl)
                      n1915 = In Range and Coerce(upper limit="Limit Max (MHz)", x=w8138, lower limit="Limit Min (MHz)") -> (In Range?=w8131:bool)  [unwired: 1 out]
                      n1916 = Not(x="Limits Enable") -> (.not. x?=w8130:bool)
                      n1917 = Or(x=w8131, y=w8130) -> (x .or. y?=w8132:bool)
                      n1918 = case shown="True" w8132 {
                        tunnel: w8139 -> [_ w8172]
                        tunnel: w8138 -> [_ w8163]
                        tunnel: w8128 -> [_ w8170]
                        tunnel: w8137 -> [_ w8169]
                        tunnel: w8126 -> [_ w8168]
                        tunnel: w8136 -> [_ w8167]
                        tunnel: w8121 -> [_ w8165]
                        tunnel: w8120 -> [_ w8164]
                        frame #0 {
                        }
                        frame #1 {
                          n1919 = local read "BD 1 Frequency 3 (MHz)"() -> (w8171:dbl)
                          n1920 = local read "BD 2 Frequency 3 (MHz)"() -> (w8166:dbl)
                          n1921 = local write "Trap Delta (MHz)"(w8163) -> ()
                          n1922 = property on="Initial delta (MHz)" class="DigNum (strict)"("Val(Sgnl)"=w8163) -> ()  [unwired: 2 in, 2 out]
                          n1923 = call "set RF board frequency - interlace.vi"("Board 2 Frequency Limits"=w8164, "Board 1 Frequency Limits"=w8165, "FPGA VI Reference In"=w8172, "Board 2 Frequency 3 (MHz)"=w8166, "Board 1 Frequency 3 (MHz)"=w8171, "Board 2 Frequency 2 (MHz)"=w8167, "Board 2 Frequency 1 (MHz)"=w8168, "Board 1 Frequency 2 (MHz)"=w8169, "Board 1 Frequency 1  (MHz)"=w8170) -> ()  [unwired: 1 in, 2 out]